vi "TA Main - PID.vi"   [LabVIEW 2019]
doc: "This example demonstrates how to acquire a continuous amount of data (Waveform) using the DAQ device's internal clock. It also shows how to synchronize two devices for different device families (E Series, S Series, M Series, X Series, DSA, and SC Express), to simultaneously acquire the data.\n\nFor instructions on how to connect your signals to the DAQ device, refer to your device documentation."
uses:
  Program Files/National Instruments/LabVIEW 2019/examples/Instrument IO/Serial/support/Serial - Settings.ctl
  <vilib>/addons/control/pid/autopid.llb/PID autotuning parameters (adv).ctl
  <vilib>/Utility/error.llb/DialogType.ctl
  <vilib>/DAQmx/read.llb/DAQmx Read (Analog 1D Wfm NChan NSamp).vi
  <vilib>/DAQmx/write.llb/DAQmx Write (Analog 1D DBL 1Chan NSamp).vi
  <vilib>/Instr/_visa.llb/VISA Configure Serial Port (Instr).vi
  <vilib>/DAQmx/configure/timing.llb/DAQmx Timing (Sample Clock).vi
  <vilib>/DAQmx/miscellaneous.llb/DAQmx Fill In Error Info.vi
  <resource>/objmgr/daqmx.rc
  <vilib>/addons/control/pid/NI_PID_autopid.lvlib
types:
  T1 = cluster{"SCD30 CO2":dbl, "SCD30 Temp (C)":dbl, "SCD30 RH (%)":dbl, "BME680 Temp (C) ":dbl, "BME680 Presssure (hPa)":dbl, "BME680 RH (%) ":dbl, "BME680 Gas (KOhms)":dbl}
  T2 = cluster{"Frequency":dbl, "Voltage (V)":dbl, "Signal type":enum16{"Sine Wave", "Triangle Wave", "Square Wave", "Sawtooth Wave"}, "Square wave duty cycle (%)":dbl, "Offset (V)":dbl, "DC shift":bool}
  T3 = cluster{"Voltage channel name":string, "Shunt channel name":string}
  T4 = cluster{"Active channel":string, "Ref channel":string}
  T5 = cluster{"X":dbl, "Y":dbl, "R":dbl, "θ":dbl, "Amp":dbl, "dt":dbl, "Active channel":string, "Ref channel":string}
  T6 = typedef "DialogType.ctl" = u16
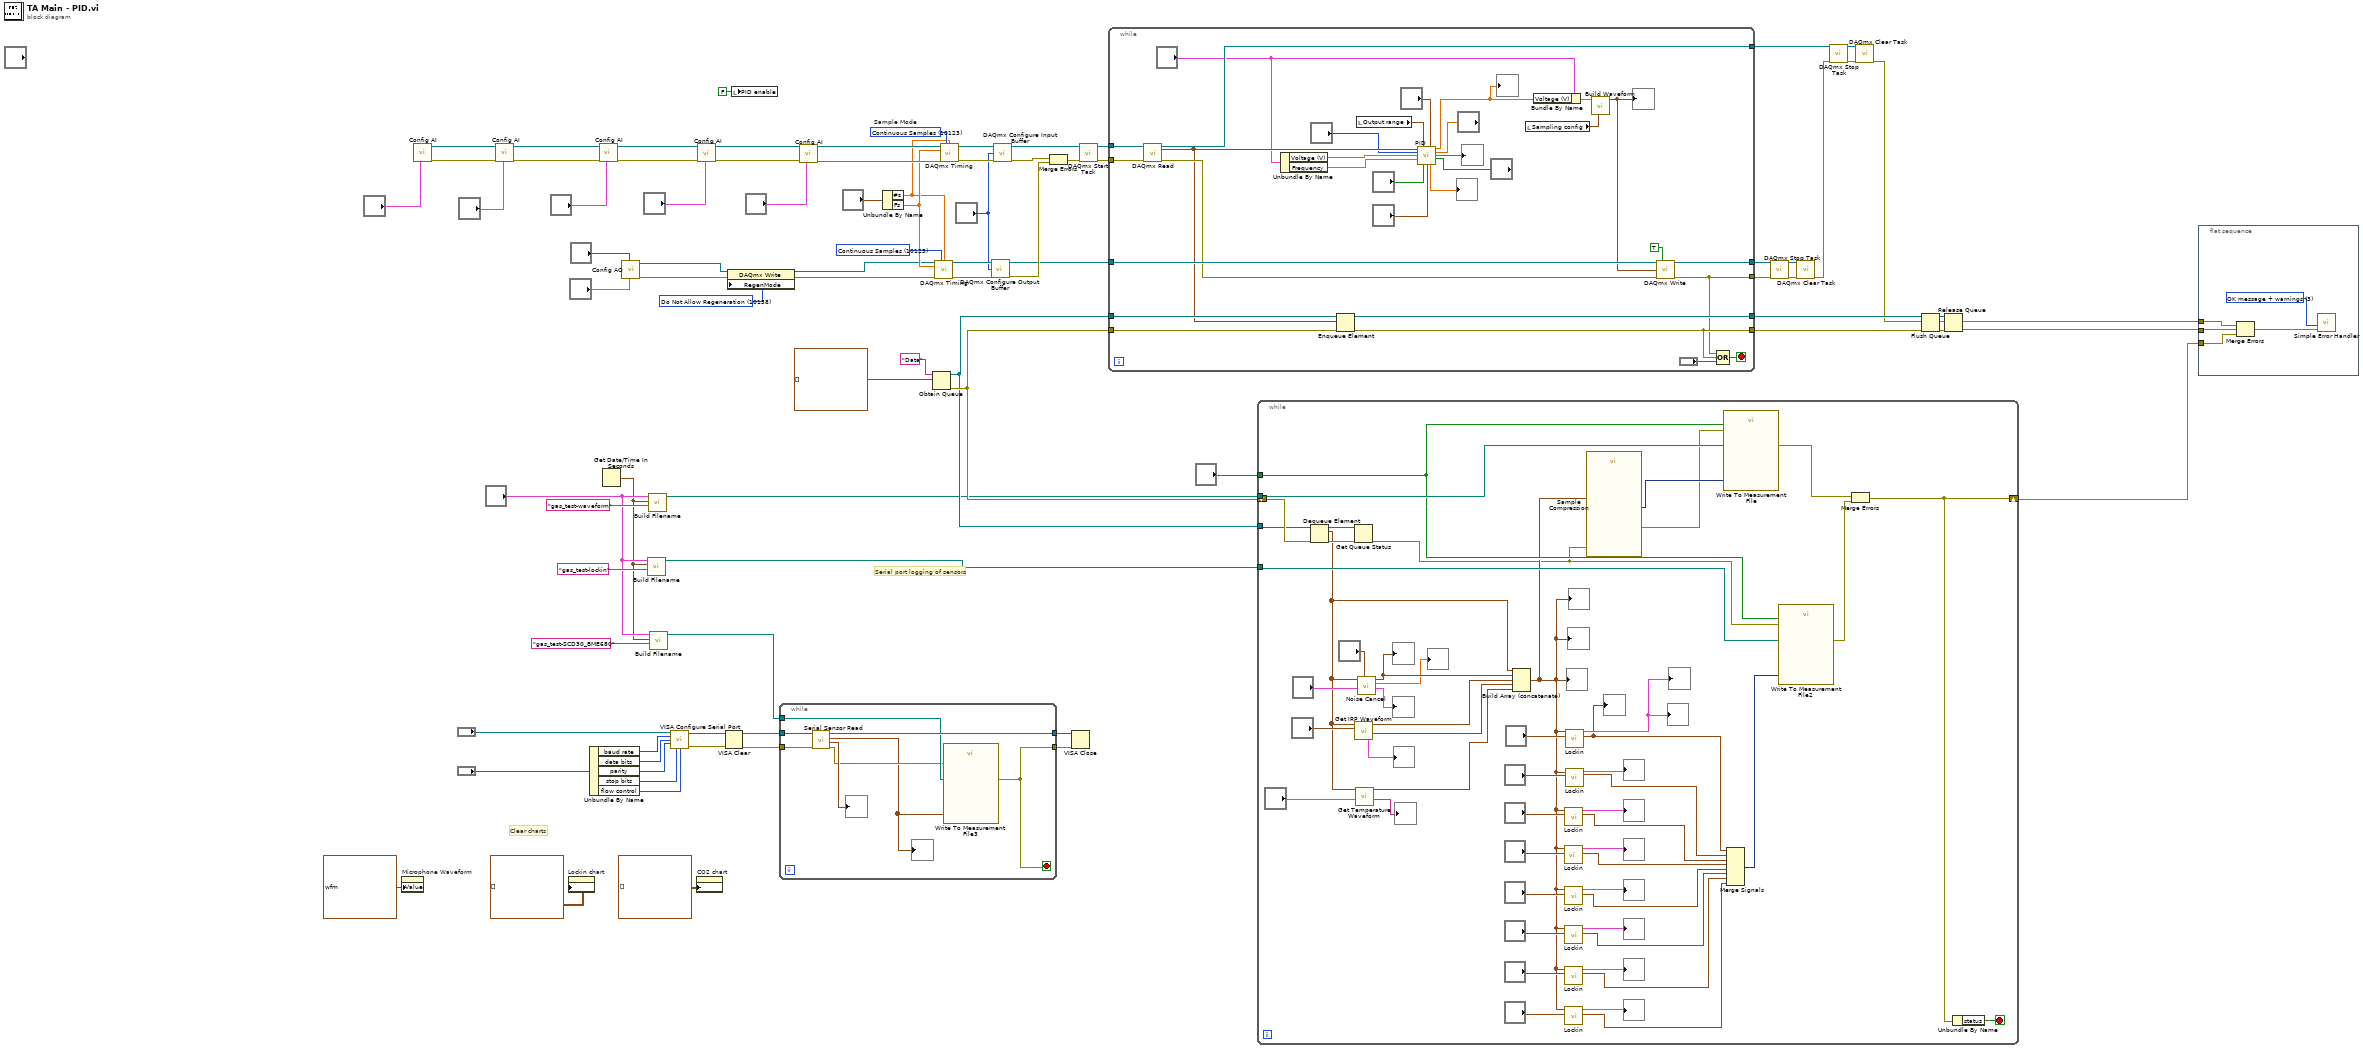
[diagram p0: block diagram]
diagram:
  w8 = 10158 items=["Allow Regeneration"=10097, "Do Not Allow Regeneration"=10158] ("RegenMode")
  w32 = 10123 items=["Finite Samples"=10178, "Continuous Samples"=10123, "Hardware Timed Single Point"=12522] ("sample mode")
  w82 = 10123 items=["Finite Samples"=10178, "Continuous Samples"=10123, "Hardware Timed Single Point"=12522]  # Sample Mode
  # "Clear charts"
  # "Serial port logging of sensors"
  n1 = property on="Microphone Waveform" class="WFGraph (strict)"("Value"=waveform(dbl)[] [{"t0"=timestamp(3651561790.263236 s since 1904-01-01), "dt"=0.001, "Y"=array[2000 elements], "attributes"=variant("NI_ChannelName"=variant(string "Mic Active"), "NI_UnitDescription"=variant(string "Volts"))}, {"t0"=timestamp(3651561790.263247 s since 1904-01-01), "dt"=0.001, "Y"=array[2000 elements], "attributes"=variant("NI_ChannelName"=variant(string "Mic Ref"), "NI_UnitDescription"=variant(string "Volts"))}, {"t0"=timestamp(3651561790.263258 s since 1904-01-01), "dt"=0.001, "Y"=array[2000 elements], "attributes"=variant("NI_ChannelName"=variant(string "Diode Heater"), "NI_UnitDescription"=variant(string "Volts"))}, {"t0"=timestamp(3651561790.263269 s since 1904-01-01), "dt"=0.001, "Y"=array[2000 elements], "attributes"=variant("NI_ChannelName"=variant(string "Diode Amb"), "NI_UnitDescription"=variant(string "Volts"))}, {"t0"=timestamp(3651561790.26328 s since 1904-01-01), "dt"=0.001, "Y"=array[2000 elements], "attributes"=variant("NI_ChannelName"=variant(string "Heater Shunt"), "NI_UnitDescription"=variant(string "Volts"))}, {"t0"=timestamp(3651561790.2632914 s since 1904-01-01), "dt"=0.001, "Y"=array[2000 elements], "attributes"=variant("NI_ChannelName"=variant(string "Heater V"), "NI_UnitDescription"=variant(string "Volts"))}, {"t0"=timestamp(3651561790.263247 s since 1904-01-01), "dt"=0.001, "Y"=array[2000 elements], "attributes"=variant("NI_ChannelName"=variant(string "Mic Diff"), "NI_UnitDescription"=variant(string "Volts"))}, {"t0"=timestamp(3651561790.26328 s since 1904-01-01), "dt"=0.001, "Y"=array[2000 elements], "attributes"=variant("NI_ChannelName"=variant(string "Heater Current"), "NI_UnitDescription"=variant(string "Amps"))}] ("Waveform")) -> ()  [unwired: 2 in, 2 out]
  n2 = call "Config AI.vi"("Channel config"="?") -> ("error out"=w81:errorcluster, "task out"=w80:refnum<k21>)  [unwired: 9 in]
  n3 = call "Config AI.vi"("Channel config"="?", "error in"=w81, "task in"=w80) -> ("error out"=w38:errorcluster, "task out"=w37:refnum<k21>)  [unwired: 7 in]
  n4 = property on="Lockin chart" class="WFChart (strict)"("History Data"=waveform(dbl)[][] []) -> ()  [unwired: 2 in, 2 out]
  n5 = Unbundle By Name("?") -> ("baud rate"=w53:u32, "data bits"=w52:u16, "parity"=w51:enum16{"None", "Odd", "Even", "Mark", "Space"}, "stop bits"=w50:u16, "flow control"=w49:u16)
  n6 = call "Config AI.vi"("Channel config"="?", "error in"=w38, "task in"=w37) -> ("error out"=w69:errorcluster, "task out"=w68:refnum<k21>)  [unwired: 7 in]
  n7 = Get Date/Time In Seconds() -> (seconds since 1Jan1904=w56:timestamp)
  n8 = call "Config AO.vi"("Channel config"="?", "Output range"="?") -> ("error out"=w10:errorcluster, "task out"=w12:refnum<k21>)  [unwired: 8 in]
  n9 = call "Build Filename.vi"("Test type"="gas_test-lockin" ("File Descriptor"), "time stamp"=w56, "File config"="?") -> ("appended path"=w59:path)  [unwired: 8 in]
  n10 = call "Build Filename.vi"("Test type"="gas_test-waveform" ("File type"), "time stamp"=w56, "File config"="?") -> ("appended path"=w61:path)  [unwired: 8 in]
  n11 = call "Build Filename.vi"("Test type"="gas_test-SCD30_BME680" ("File Descriptor"), "time stamp"=w56, "File config"="?") -> ("appended path"=w42:path)  [unwired: 8 in]
  n12 = call-poly "VISA Configure Serial Port"("VISA resource name"="?", "baud rate (9600)"=w53, "data bits (8)"=w52, "parity (0:none)"=w51, "stop bits (10: 1 bit)"=w50, "flow control (0:none)"=w49) -> ("VISA resource name out"=w47:refnum<visa-resource-name>, "error out"=w48:errorcluster)  [unwired: 3 in, 5 out]
  n13 = property on="CO2 chart" class="WFChart (strict)"("History Data"=waveform(dbl)[][] []) -> ()  [unwired: 2 in, 2 out]
  n14 = call "Config AI.vi"("Channel config"="?", "error in"=w69, "task in"=w68) -> ("error out"=w35:errorcluster, "task out"=w34:refnum<k21>)  [unwired: 7 in]
  n15 = VISA Clear(VISA resource name=w47, error in (no error)=w48) -> (VISA resource name out=w46:refnum<visa-resource-name>, error out=w45:errorcluster)
  n16 = property class="DAQmx Write"(reference=w12, error in=w10, "RegenMode"=w8) -> (reference out=w11:refnum<k21>, error out=w9:errorcluster)
  n17 = local write "PID enable"(FALSE ("PID enable")) -> ()
  n18 = while {
    tunnel: w46 -> [w92]
    tunnel: w45 -> [w91]
    tunnel: [w86] -> w44
    tunnel: [w90] -> w43
    tunnel: w42 -> [w88]
    stop <- w86 stop-if-true
    n19 = call "Serial Sensor Read.vi"("error in (no error)"=w91, "VISA resource name"=w92) -> ("error out"=w87:errorcluster, "Readings"=→"?":T1, "appended array"=w85:waveform(dbl)[], "VISA resource name out"=w90:refnum<visa-resource-name>)  [unwired: 6 in]
    "?" <- w85
    n20 = call "Write To Measurement File3"("Signals"=w85, "error in (no error)"=w87, "Filename"=w88) -> ("error out"=w86:errorcluster)  [unwired: 14 in, 2 out]
  }
  n21 = call "Config AI.vi"("Channel config"="?", "error in"=w35, "task in"=w34) -> ("error out"=w31:errorcluster, "task out"=w30:refnum<k21>)  [unwired: 7 in]
  n22 = Unbundle By Name("?") -> ("#s"=w7:dbl, "Fs"=w29:dbl)
  n23 = Obtain Queue(name (unnamed)="Data" ("名前（名前なし）"), element data type=waveform(dbl)[] [] ("data")) -> (queue out=w72:refnum<queue>, error out=w73:errorcluster)  [unwired: 3 in, 1 out]
  n24 = call-poly <vilib>:"DAQmx Timing.vi"("task/channels in"=w11, "sample mode"=w32, "samples per channel"=w7, "rate"=w29, "error in"=w9) -> ("task out"=w6:refnum<k21>, "error out"=w5:errorcluster)  [unwired: 9 in]
  n25 = call-poly <vilib>:"DAQmx Timing.vi"("task/channels in"=w30, "sample mode"=w82, "samples per channel"=w7, "rate"=w29, "error in"=w31) -> ("task out"=w13:refnum<k21>, "error out"=w16:errorcluster)  [unwired: 9 in]
  n26 = call <vilib>:"DAQmx Configure Output Buffer.vi"("task/channels in"=w6, "buffer size (in samples per channel)"="?", "error in"=w5) -> ("task out"=w2:refnum<k21>, "error out"=w3:errorcluster)  [unwired: 11 in]
  n27 = call <vilib>:"DAQmx Configure Input Buffer.vi"("task/channels in"=w13, "buffer size (in samples per channel)"="?", "error in"=w16) -> ("task out"=w14:refnum<k21>, "error out"=w15:errorcluster)  [unwired: 11 in]
  n28 = Merge Errors(w15, w3) -> (w28:errorcluster)
  n29 = VISA Close(VISA resource name=w43, error in (no error)=w44) -> ()  [unwired: 1 out]
  n30 = call <vilib>:"DAQmx Start Task.vi"("task/channels in"=w14, "error in"=w28) -> ("task out"=w27:refnum<k21>, "error out"=w26:errorcluster)  [unwired: 12 in]
  n31 = while {
    tunnel: [w122] -> w77
    tunnel: [w118] -> w76
    tunnel: w72 -> [w121]
    tunnel: w73 -> [w120]
    tunnel: w27 -> [w117]
    tunnel: w26 -> [w116]
    tunnel: w2 -> [w115]
    tunnel: [w114] -> w24
    tunnel: [w109] -> w21
    tunnel: [w110] -> w20
    stop <- w123 stop-if-true
    n32 = call-poly <vilib>:"DAQmx Read.vi"("task/channels in"=w117, "error in"=w116) -> ("task out"=w114:refnum<k21>, "data"=w107:waveform(dbl)[], "error out"=w111:errorcluster)  [unwired: 11 in]
    n33 = Unbundle By Name("?") -> ("Voltage (V)"=w105:dbl, "Frequency"=w106:dbl)
    n34 = Enqueue Element(queue=w121, element=w107, error in (no error)=w120) -> (queue out=w122:refnum<queue>, error out=w118:errorcluster)  [unwired: 1 in, 1 out]
    n35 = local read "Output range"() -> (w99:cluster{"output high":dbl, "output low":dbl})
    n36 = call "PID.vi"("array"=w107, "output range"=w99, "autotuning parameters"="?", "index"="?", "Setpoint"="?", "manual control"=w105, "Frequency"=w106, "reinitialize? (F)"="?", "auto? (F)"="?", "PID gains"="?") -> ("output"=w95:dbl, "Channel name"=→"?":string, "Input"=→"?":dbl)  [unwired: 2 in, 1 out]
    "?" <- w95
    n37 = local read "Sampling config"() -> (w113:cluster{"Fs":dbl, "#s":dbl})
    n38 = Bundle By Name(cluster="?", "Voltage (V)"=w95) -> (w96:T2)
    n39 = call "Build Waveform.vi"("sampling config"=w113, "Config"=w96) -> ("Waveform"=w112:waveform(dbl))  [unwired: 8 in, 1 out]
    "?" <- w112
    n40 = call-poly <vilib>:"DAQmx Write.vi"("task/channels in"=w115, "auto start"=TRUE, "data"=w112, "error in"=w111) -> ("task out"=w110:refnum<k21>, "error out"=w109:errorcluster)  [unwired: 9 in, 1 out]
    n41 = Compound Arithmetic op=OR(w109, w118, "?") -> (w123:bool)
  }
  n42 = while {
    tunnel: w72 -> [w175]
    shift-right: [w167] -> w71
    shift-left: w73 -> [w176]
    tunnel: w61 -> [w174]
    tunnel: "?" -> [w171]
    tunnel: w59 -> [w170]
    stop <- w163 stop-if-true
    n43 = Dequeue Element(queue=w175, error in (no error)=w176) -> (queue out=w172:refnum<queue>, element=w135:waveform(dbl)[], error out=w173:errorcluster)  [unwired: 1 in, 1 out]
    n44 = Get Queue Status(queue=w172, error in (no error)=w173) -> (error out=w128:errorcluster)  [unwired: 1 in, 7 out]
    n45 = call "Get IRP Waveform.vi"("Channel config"="?", "array"=w135) -> ("Power waveform out"=w134:waveform(dbl), "Current waveform out"=w143:waveform(dbl), "Channel names"=→"?":T3)  [unwired: 6 in, 1 out]
    n46 = call "Get Temperature Waveform.vi"("Config"="?", "array"=w135) -> ("Channel name"=→"?":string, "waveform out"=w133:waveform(dbl))  [unwired: 8 in]
    n47 = call "Noise Cancel.vi"("Filter config"="?", "Config"="?", "array"=w135) -> ("Channel names"=→"?":T4, "Noise estimate (mVrms)"=→"?":dbl, "waveform out"=w165:waveform(dbl))  [unwired: 6 in]
    "?" <- w165
    n48 = Build Array (concatenate)(w135, w165, w143, w134, w133) -> (w130:waveform(dbl)[])
    "?" <- w130
    "?" <- w130
    "?" <- w130
    n49 = call "Lockin.vi"("Config"="?", "array"=w130) -> ("Output waveform"=w159:waveform(dbl)[], "Lockin output"=→"?":T5)  [unwired: 8 in]
    n50 = call "Lockin.vi"("Config"="?", "array"=w130) -> ("Output waveform"=w160:waveform(dbl)[], "Lockin output"=→"?":T5)  [unwired: 8 in]
    n51 = call "Lockin.vi"("Config"="?", "array"=w130) -> ("Output waveform"=w158:waveform(dbl)[], "Lockin output"=→"?":T5)  [unwired: 8 in]
    n52 = call "Lockin.vi"("Config"="?", "array"=w130) -> ("Output waveform"=w157:waveform(dbl)[], "Lockin output"=→"?":T5)  [unwired: 8 in]
    n53 = call "Lockin.vi"("Config"="?", "array"=w130) -> ("Output waveform"=w139:waveform(dbl)[], "Lockin output"=→"?":T5)  [unwired: 8 in]
    n54 = call "Lockin.vi"("Config"="?", "array"=w130) -> ("Output waveform"=w126:waveform(dbl)[], "Lockin output"=→"?":T5)  [unwired: 8 in]
    n55 = call "Lockin.vi"("Config"="?", "array"=w130) -> ("Output waveform"=w145:waveform(dbl)[], "Lockin output"=→"?" →"?":T5)  [unwired: 8 in]
    "?" <- w145
    n56 = call "Lockin.vi"("Config"="?", "array"=w130) -> ("Output waveform"=w161:waveform(dbl)[], "Lockin output"=→"?":T5)  [unwired: 8 in]
    n57 = call "Sample Compression"("error in (no error)"=w128, "Signals"=w130) -> ("error out"=w127:errorcluster, "Mean"=w129:dynamicdata)  [unwired: 7 in, 1 out]
    n58 = call "Write To Measurement File"("Signals"=w129, "Enable"=w171, "error in (no error)"=w127, "Filename"=w174) -> ("error out"=w168:errorcluster)  [unwired: 13 in, 2 out]
    n59 = Merge Signals(w145, w161, w160, w159, w158, w157, w139, w126) -> (w156:dynamicdata)
    n60 = call "Write To Measurement File2"("Signals"=w156, "Enable"=w171, "error in (no error)"=w128, "Filename"=w170) -> ("error out"=w169:errorcluster)  [unwired: 13 in, 2 out]
    n61 = Merge Errors(w168, w169) -> (w167:errorcluster)
    n62 = Unbundle By Name(w167) -> ("status"=w163:bool)
  }
  n63 = call <vilib>:"DAQmx Stop Task.vi"("task/channels in"=w20, "error in"=w21) -> ("task out"=w22:refnum<k21>, "error out"=w23:errorcluster)  [unwired: 12 in]
  n64 = call <vilib>:"DAQmx Clear Task.vi"("task in"=w22, "error in"=w23) -> ("error out"=w19:errorcluster)  [unwired: 13 in]
  n65 = call <vilib>:"DAQmx Stop Task.vi"("task/channels in"=w24, "error in"=w19) -> ("task out"=w83:refnum<k21>, "error out"=w84:errorcluster)  [unwired: 12 in]
  n66 = call <vilib>:"DAQmx Clear Task.vi"("task in"=w83, "error in"=w84) -> ("error out"=w25:errorcluster)  [unwired: 13 in]
  n67 = Flush Queue(queue=w77, error in (no error)=w76) -> (queue out=w78:refnum<queue>, error out=w79:errorcluster)  [unwired: 1 out]
  n68 = Release Queue(queue=w78, error in (no error)=w79) -> (error out=w75:errorcluster)  [unwired: 1 in, 2 out]
  n69 = flat-sequence {
    tunnel: w25 -> [w181]
    tunnel: w75 -> [w180]
    tunnel: w71 -> [w177]
    frame #0 {
      w179 = T6 3 items=["no dialog", "OK message", "continue or stop message", "OK message + warnings", "continue/stop + warnings"] ("type of dialog (OK msg:1)")
      n70 = Merge Errors(w181, w180, w177) -> (w178:errorcluster)
      n71 = call <vilib>:"Simple Error Handler.vi"("type of dialog (OK msg:1)"=w179, "error in (no error)"=w178) -> ()  [unwired: 3 in, 5 out]
    }
  }
